vi "Example_DAQ.vi"() -> ()   [LabVIEW 2013]
uses:
  Instance           6 19Saved   Example_DAQ .vi
  <vilib>/Signadyne/DAQ/base/DAQread_TDC.vi
panel:
  in  "edge":enum32{"Rising Edge", "Falling Edge"}(ring)
  out "Data Points":i32=1000000
  in  "slot":i32=4
  in  "Threshold (V)":dbl
  out "Waveform Chart":i32(graph)=1063830
  out "Rate Counter":i32=1063830
  out "Loop Count":i32=2
  out "Rate Counter":i32=1063830
  out "Config  Status":errorcluster
  in  "DAQtimeout":i32=2000
  in  "DAQpoints":i32=1000
  out "TimeStampData":u64[](array[numeric])
  out "DAQ Timestamp Counter":i32=2999744
  in  "Channel / DAQ":i32 min=0 max=7 step=1
  out "Close Status":errorcluster
  in  "Stop Aquisition":bool
  in  "Part Number":string="SD-PXE-TDC-H0002"
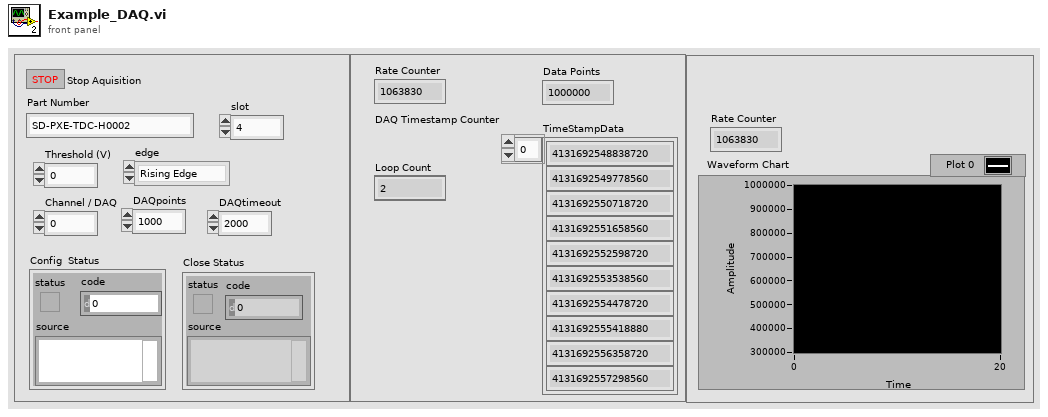
[diagram p1: front panel]
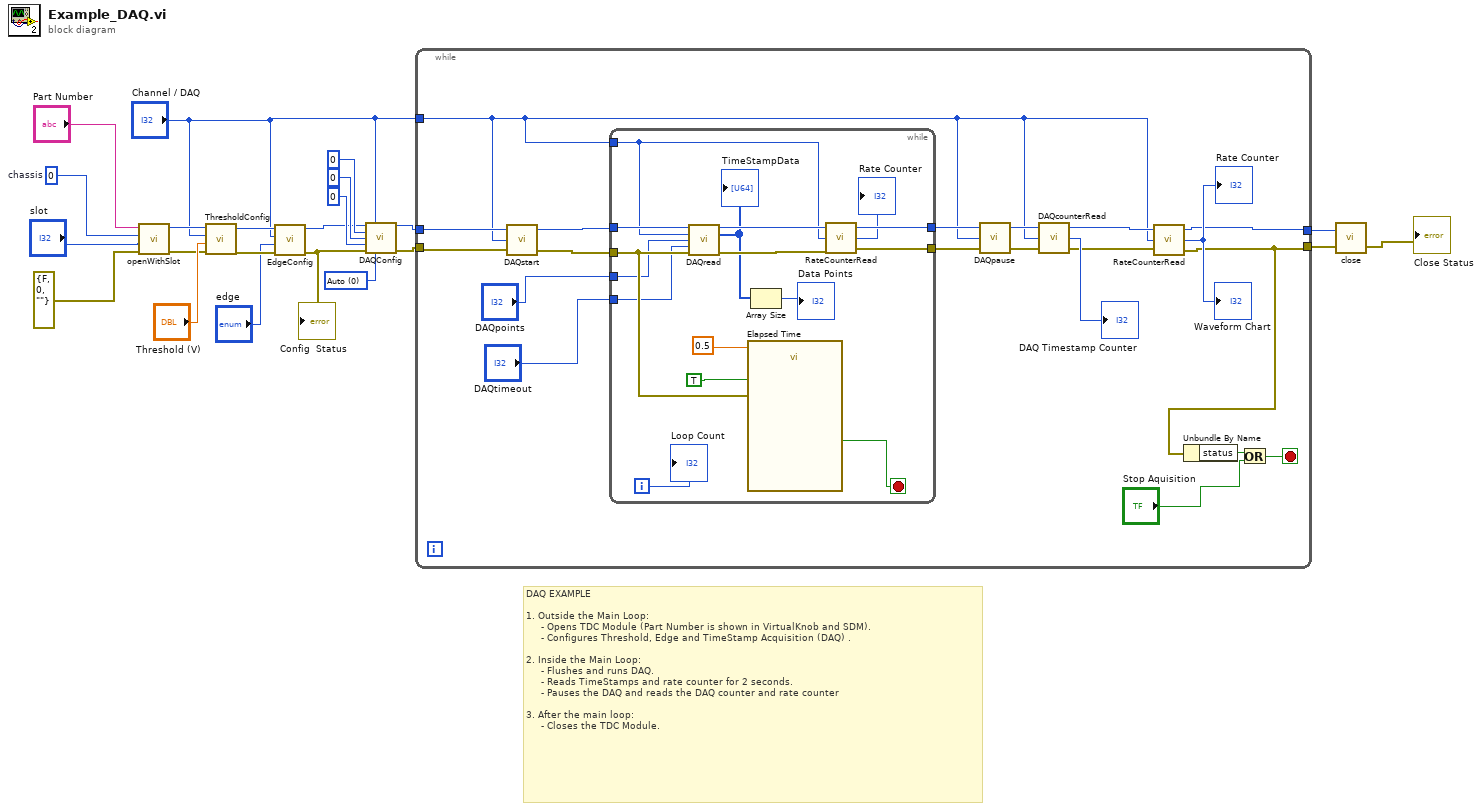
[diagram p0: block diagram]
diagram:
  w1 = 0 items=["Auto", "VI/HVI", "External"] ("triggerMode")
  w14 = 0  # chassis
  # "DAQ EXAMPLE\n\n1. Outside the Main Loop:\n     - Opens TDC Module (Part Number is shown in VirtualKnob and SDM).\n     - Configures Threshold, Edge and TimeStamp Acquisition (DAQ) .\n\n2. Inside the Main Loop:\n     - Flushes and runs DAQ.\n     - Reads TimeStamps and rate counter for 2 seconds.\n     - Pauses the DAQ and reads the DAQ counter and rate counter\n\n3. After the main loop:\n     - Closes the TDC Module."
  n1 = call <vilib>:"openWithSlot.vi"("errorIn"=errorcluster {"status"=FALSE, "code"=0, "source"=""}, "nSlot"="slot", "nChassis"=w14, "partNumber"="Part Number") -> ("errorOut"=w11:errorcluster, "moduleID"=w10:i32)  [unwired: 2 in]
  n2 = call <vilib>:"ThresholdConfig.vi"("errorIn"=w11, "threshold"="Threshold (V)", "nChannel"="Channel / DAQ", "moduleID"=w10) -> ("errorOut"=w22:errorcluster, "moduleIDout"=w21:i32)  [unwired: 2 in]
  n3 = call <vilib>:"EdgeConfig.vi"("errorIn"=w22, "edge"="edge", "nChannel"="Channel / DAQ", "moduleID"=w21) -> ("errorOut"=w4:errorcluster, "moduleIDout"=w2:i32)  [unwired: 2 in]
  "Config  Status" <- w4
  n4 = call <vilib>:"DAQConfig.vi"("moduleID"=w2, "nDAQ"="Channel / DAQ", "DAQpointsPerCycle"=0, "cycles"=0, "prescaler"=0, "errorIn"=w4, "triggerMode"=w1) -> ("moduleIDout"=w9:i32, "errorOut"=w8:errorcluster)  [unwired: 7 in]
  n5 = while {
    tunnel: w8 -> [w38]
    tunnel: [w30] -> w17
    tunnel: [w24] -> w18
    tunnel: "Channel / DAQ" -> [w23]
    tunnel: w9 -> [w37]
    stop <- w25 stop-if-true
    n6 = call <vilib>:"DAQstart.vi"("errorIn"=w38, "nDAQ"=w23, "moduleID"=w37) -> ("errorOut"=w42:errorcluster, "moduleIDout"=w40:i32)  [unwired: 1 in]
    n7 = while {
      tunnel: w40 -> [w50]
      tunnel: [w55] -> w41
      tunnel: w23 -> [w44]
      tunnel: w42 -> [w47]
      tunnel: [w54] -> w39
      tunnel: "DAQtimeout" -> [w46]
      tunnel: "DAQpoints" -> [w45]
      i -> [w52]
      stop <- w56 stop-if-true
      n8 = call-poly <vilib>:"DAQread.vi"("moduleID"=w50, "nDAQ"=w44, "DAQpoints"=w45, "TimeOut"=w46, "errorIn"=w47) -> ("moduleIDout"=w49:i32, "DAQdata"=w43:i64[], "errorOut"=w48:errorcluster)  [unwired: 8 in]
      "TimeStampData" <- w43
      n9 = call "Elapsed Time"("Time Target (s)"=0.5 ("Delay Time (s)"), "Auto Reset"=TRUE, "error in (no error)"=w47) -> ("Time has Elapsed"=w56:bool)  [unwired: 9 in, 7 out]
      n10 = Array Size(array=w43) -> (size(s)=→"Data Points":i32)
      n11 = call <vilib>:"RateCounterRead.vi"("errorIn"=w48, "nChannel"=w44, "moduleID"=w49) -> ("errorOut"=w54:errorcluster, "countRate"=→"Rate Counter":i32, "moduleIDout"=w55:i32)
      "Loop Count" <- w52
    }
    n12 = call <vilib>:"DAQpause.vi"("errorIn"=w39, "nDAQ"=w23, "moduleID"=w41) -> ("errorOut"=w35:errorcluster, "moduleIDout"=w34:i32)  [unwired: 1 in]
    n13 = call <vilib>:"DAQcounterRead.vi"("errorIn"=w35, "nDAQ"=w23, "moduleID"=w34) -> ("errorOut"=w31:errorcluster, "DAQcounts"=→"DAQ Timestamp Counter":i32, "moduleIDout"=w32:i32)
    n14 = call <vilib>:"RateCounterRead.vi"("errorIn"=w31, "nChannel"=w23, "moduleID"=w32) -> ("errorOut"=w24:errorcluster, "countRate"=→"Rate Counter" →"Waveform Chart":i32, "moduleIDout"=w30:i32)
    n15 = Unbundle By Name(w24) -> ("status"=w27:bool)
    n16 = Or(x=w27, y="Stop Aquisition") -> (x .or. y?=w25:bool)
  }
  n17 = call <vilib>:"close.vi"("errorIn"=w18, "moduleID"=w17) -> ("errorOut"=→"Close Status":errorcluster)  [unwired: 1 in]
